vi "UHR-Fleezers Control (host) - Avogadro v1.vi"() -> ()   [LabVIEW 2014] (continued)
  out "GI Late Counter 2":u8
  in  "Phase adj. (GI) 2":i16=1
  out "GI relative phase 2":i16
  in  "+ phase (GI) 2":bool
  in  "Initial Phase Adjustment (GI) 2":i16=-274
  in  "- phase (GI) 2":bool
  in  "Green FB Gains":T14={"proportional gain (Kc)"=10, "integral gain (Kc*Ts/Ti)"=5, "derivative gain (Kc*Td/Ts)"=0}
  in  "Green int current ON count adj":u32=150
  in  "- phase (GI)":bool
  in  "Initial Phase Adjustment (GI)":i16=-28
  in  "+ phase (GI)":bool
  out "GI relative phase":i16
  in  "Phase adj. (GI)":i16=1
  out "GI Late Counter":u8
  out "Green AI Late Counter":u8
  out "MCL Scan":cluster{"Begin (V)":dbl, dbl, dbl[]}(graph)
  out "MCL Scan 2":cluster{"Begin (V)":dbl, dbl, dbl[]}(graph)
  out "Red laser intensity (V)":dbl
  out "Red AI Count":u16=600
  in  "Initial Phase Adjustment (RI)":i16=25
  out "RI Late Counter":u8
  in  "Red FB Gains":T14={"proportional gain (Kc)"=10, "integral gain (Kc*Ts/Ti)"=5, "derivative gain (Kc*Td/Ts)"=0}
  in  "Phase adj. (RI)":i16=20
  out "RI relative phase":i16
  in  "+ phase (RI)":bool
  in  "- phase (RI)":bool
  in  "Blue Laser Modulation Mode":string(combo)
  out "Digital Modulation":bool
  out "Analog Modulation":bool
  out "Laser On":bool
  in  "Get Blue Laser State":bool
  out "Blue laser intensity (V)":dbl
  out "Relative phase (BI AO)":i16
  out "Relative phase (BI DO)":i16
  out "Late Counter (BI DO)":u8
  out "Late Counter (BI AO)":u8
  in  "Initial Phase Adjustment (BI DO)":i16=65
  in  "Initial Phase Adjustment (BI AO)":i16
  in  "Phase adj. (BI AO)":i16=20
  in  "+ phase (BI AO)":bool
  in  "- phase (BI AO)":bool
  in  "Blue int AO ON count adjust":u16=150
  in  "Blue FB Gains":T14={"proportional gain (Kc)"=10, "integral gain (Kc*Ts/Ti)"=5, "derivative gain (Kc*Td/Ts)"=0}
  in  "- phase (BI DO)":bool
  in  "+ phase (BI DO)":bool
  in  "Phase adj. (BI DO)":i16=20
  out "Blue AI Count":u16=600
  in  "Delay (ms)":i32=500
  in  "Send string\nto Blue Laser":bool
  in  "command string":string
  out "command string sent":string="sames 0"
  out "read blue buffer":string
  out "Blue Error Out":errorcluster={"status"=TRUE, "code"=-1073807346, "source"="VISA Write in serial write macro.vi->UHR-Fleezers Control (host) - Avogadro v1.vi"}
  in  "VISA resource name":refnum<visa-resource-name>="Blue-Laser-COM7"
  in  "Blue Laser Modulation\nPower (mW)":string="80"
  in  "Blue Laser Power (mW)\n(Constant Power Mode)":string="70"
  in  "Flip X Sign":bool=TRUE
  in  "Trap Position FIFO Depth":u32=300000 format="%.0p"
  in  "# Samples/trap":u32=20000
  out "Trap AI Elements/DMA read":u32=320000 format="%.0p"
  out "Ave. Rate (Hz)":dbl=200000.0 format="%#_6p"
  out "FIFO El. Rem.":u32=3 format="%.0p"
  in  "Phase adj. (AI1)":i16=10
  out "Relative phase (AI1)":i16=-170
  in  "+ phase (AI1)":bool
  in  "- phase (AI1)":bool
  out "Late Counter (AI1)":u8
  in  "Initial Phase Adjustment (AI1)":i16=170
  out "AI rate (Hz)":dbl=200000.0 format="%#_6p"
  in  "AI Count (ticks)":u16=200
  out "# Samples/channel":u32=40000 format="%.0p"
  in  "Trap AI FIFO Depth":u32=900000
  in  "Detector Type":string(combo)="IR-QPD + PSD + FB-QPD X position"
  in  "N Acq Sets (Traps + Fl.)":i16=2
  in  "Sets to FIFO (Traps)":T22={"Set 1"=TRUE, "Set 2"=TRUE, "Set 3"=FALSE}
  in  "FPGA Ave.":dbl=1.0 min=1.0 step=1.0
  out "Ave. Period (s)":dbl=5e-06 format="%#_6p"
  out "DMA Update Period (s)":dbl=0.2
  out "FPGA Averaging":bool
  out "Trap Sets":u32=2
  out "Counts/DMA":dbl=8000000.0 format="%#_6p"
  out "Trap Pos FIFO El Remaining":u32=2905 format="%.0p"
  out "Trap Pos Elements/DMA read":u32=200000 format="%.0p"
  out "Trap AI FIFO Timeout":u16
  out "Trap Pos FIFO Timeout":u16
  out "error out":errorcluster
  out "error out 2":errorcluster
  in  "Piezo trap y\noffset (V)":dbl=0.6709036530655844
  in  "Piezo trap x\noffset (V)":dbl=-6.361797973205792
  in  "Piezo Trap Y cal (nm/V)":dbl=279.6
  in  "Piezo Trap X cal (nm/V)":dbl=362.7
  in  "Bottom  1 Harvard Syringe Pump Serial Port":refnum<visa-resource-name>="Bottom-Pump1-COM5"
  in  "Center Harvard Syringe Pump Serial Port":refnum<visa-resource-name>="Central-Pump2-COM6"
  in  "Lost Tether Alarm Threshold (pN)":dbl=0.5
  in  "AOM X Cal (nm/MHz)":dbl=203.0
  in  "MCL X Cal (nm/V)":dbl=739.5
  out "X RF Amplitude Limits (%)":T23={"Minimum"=0.0, "Maximum"=50.0, "Increment"=1.0}
  out "X RF Frequency Limits (MHz)":T23={"Minimum"=60.0, "Maximum"=90.0, "Increment"=1.0}
  out "Y RF Frequency Limits (MHz)":T23={"Minimum"=0.0, "Maximum"=40.0, "Increment"=0.1}
  out "Y RF Amplitude Limits (%)":T23={"Minimum"=0.0, "Maximum"=45.0, "Increment"=1.0}
  in  "Manip. X?":bool=TRUE
  in  "Manip. Y?":bool
  in  "Force Manip Abort":bool
  out "Read cal error":errorcluster
  in  "DAQ Delay (ms)":u32=1000
  in  "Start Scan":bool
  in  "Scan axis":bool=TRUE
  in  "Osc. amp. (V)":dbl=5.0
  in  "Osc. center (V)":dbl=5.0
  in  "Osc. freq. (Hz) 2":dbl=1.0
  in  "MCL Mode":u16(ring) items=["Manual Positioning", "Sinusoidal Wave", "Linear Scan"]
  in  "Begin (V)":dbl
  in  "End (V)":dbl=10.0
  in  "N Points":dbl=20.0
  in  "Delay to Interlace (s)":dbl
  in  "Delayed Interlace Start":bool
  in  "Read Lateness and Rel Phase":bool=TRUE
  out "Vec Mean of T1 T2":dbl[](array[numeric])=[-361.2890180339416, -361.0696389052203]
  in  "Cal read wait (s)":u32=5
  out "Time tether formed":timestamp=timestamp(3534521622.0325327 s since 1904-01-01)
  in  "Sample Chamber Stage Serial Port":refnum<visa-resource-name>="Sample-Stage-COM1"
  in  "Chemyx Syringe Pump Serial Port":refnum<visa-resource-name>="ASRL3::INSTR"
  in  "Limit Min (MHz)":dbl=10.0 caption="Min (MHz)"
  in  "Limit Max (MHz)":dbl=16.0 caption="Max (MHz)"
  in  "Limits Enable":bool=TRUE caption="Enable"
  out "AI labels":string[](array[string])=["T1 Y", "T1 X", "T1 Sum", "T2 Y", "T2 X", "T2 Sum", "T1 FB X", "T1 FB Sum", "T2 FB X", "T2 FB Sum", "T3 Y/ PSD Y", "T3 X / PSD X", "T3 Sum / PSD sum"]
  in  "Save Trap Pos. Data":bool=TRUE
  in  "Lower Ch. Cap.":bool
  in  "Top 3 Harvard Syringe Pump Serial Port":refnum<visa-resource-name>="Top-Pump3-COM4"
  out "Database link":path=path "C:/Home/Bustamante Lab/Comstock-LabView-Link.udl"
  out "connection reference":T24
  out "FPGA error out":errorcluster
  out "Trigger Signal":dbl[](graph)=[1.953852737276498, 1.8613052147403675]
  in  "Fish mask thresh":dbl=0.5
  in  "Normal (on) or masked test (off)":bool=TRUE
  in  "Stop F (pN) (mask)":dbl=1.0
  in  "Osc. freq. (Hz)":dbl=0.25
  in  "Trap shift\nmethod":bool=TRUE
  in  "Pause rotation":bool
  out "Waveform Chart":dbl(graph)
  in  "Trap 2 phase shift (deg)":dbl caption="Fixed phase shift (deg)"
  in  "Radius (MHz)":dbl=2.0 min=0.0 max=10.0 step=0.1
  out "Trap trajectories":cluster{dbl[], dbl[]}[](graph)
  in  "Move in a Circle":bool
  in  "Center Y Frequency (MHz)":dbl=31.0
  in  "Stop Moving":bool
  in  "2D Motion Frequency (Hz)":dbl=0.25
  in  "2D Motion Trap Separation (MHz)":dbl=0.75 caption="Fixed distance (MHz)" min=0.0 max=10.0 step=0.1
  in  "Time step (ms)":i64=10
  in  "N steps then stop":i32
  in  "Back to start on finish?":bool=TRUE
  in  "Counterclockwise/Clockwise":bool
  out "Trap 1 sum mean":dbl=-0.0915169228862244 format="%0.2f"
  out "Trap 2 sum mean":dbl=-0.06760925671124465 format="%0.2f"
  in  "index 1":i32=3
  in  "index 2":i32
  in  "test":bool
  in  "Reset graph":bool
  in  "N steps to plot":i32=1000
  out "Waveform Graph 2":waveform(dbl)(graph)
  in  "Offset 2":dbl
  in  "mult x":dbl
  in  "Offset":dbl
  out "N data samples":dbl
  out "Initial buffer time (s)":dbl
  in  "N initial buffer elements":u16=5000
  in  "Sound ON":bool
  in  "Carrier Frequency (Hz)":dbl=300.0
  in  "number of samples/ch":i32=100000
  in  "sample mode":T25=1 items=["Finite Samples", "Continuous Samples"]
  in  "device ID":u32
  in  "sound format":T26={"sample rate (S/s)"=22050.0, "number of channels"=2, "bits per sample"=16}
  in  "Volume":dbl=1.0 format="%0.2p"
  in  "interpolation mode":u16(ring)=1 items=["coerce", "linear", "spline", "FIR filter"]
  in  "tone or data":bool
  in  "Data channel to sound":i32
  in  "Base N trap periods":u32=50
  in  "Period scale factor":dbl=4.0
  in  "Trap osc amp (MHz)":dbl=1.0
  in  "Osc trap cont.":bool
  in  "Osc traps":bool
  out "Trap OSC Period (s)":dbl=0.002
  out "Writing waveform to fpga memory":bool
  in  "Save trap pos with cal":bool=TRUE
  in  "T1 Osc Enable":bool=TRUE
  in  "T2 Osc Enable":bool=TRUE
  out "DMA remainder":u64
  out "(total save/100) /osc period remainder":u32
  out "Total save/100 remainder":u32
  out "N osc/ (total save/100)":u64=25
  out "N osc / DMA":u64=100
  out "N trap osc periods per save":u64
  out "N trap osc periods per save remainder":u64
  in  "Command":string
  out "Reply":string
  in  "Send Command":bool
  out "Preamp Error Out":errorcluster
  in  "Gain Mode":string(combo)="0"
  in  "Invert Signal":bool
  in  "Sensitivity":string(combo)="0"
  in  "Offset Current Sign":bool=TRUE
  in  "Offset Current Value":string(combo)
  in  "Offset Current":bool
  in  "Bias Voltage":bool
  in  "Bias Voltage (mV)":i32
  in  "Filter Type":string(combo)="4"
  in  "Lowpass 3dB Point":string(combo)="6"
  in  "Highpass 3dB Point":string(combo)
  in  "Filter Reset":bool
  out "Command Sent":string
  out "Gain":string(combo)="0"
  # "X"
  # "Y"
  # "Data Saving"
  # "External fluorescence triggering tests:"
  # "After"
  # "During"
  # "Trap On?"
  # "BD Flow ON?"
  # "Samp Flow ON?"
  # "Trap Trig. Fl.?"
  # "Zero It"
  # "Floor it\n(e.g., hp unwinding)"
  # "1"
  # "2"
  # "Fl. Down"
  # "Fl. Up"
  # "T1 Y"
  # "T1 X"
  # "T1 Sum"
  # "T2 Y"
  # "T2 X"
  # "T2 Sum"
  # "FB1 X"
  # "FB1 Sum"
  # "FB2 X"
  # "FB2 Sum"
  # "T3 Y"
  # "T3 X"
  # "T3 Sum"
  # "Trap Display:"
  # "APD Display:"
  # "DAQ"
  # "Trap Manipulation"
  # "Bead Calibration"
  # "MCL trap"
  # "Trap 3"
  # "Fl"
  # "Fine Motor Control"
  # "Bottom Pump (#1)"
  # "Central Sample Channels"
  # "Top Pump (#3)"
  # "Rate param is ul/h\nVolume param is ul"
  # "Chemyx Pump 2"
  # "Units: \n1 = ml/m\n2 = ml/h\n3 = ul/m\n4 = ul/h"
  # "Choose method of updating trap RF values: false is usual, true is use external loop method\n(in order to increase possible delay between X and Y signals -- to synchronize X and Y switching)"
  # "Delay to switch frequency and amplitude of boards.\nUsed to align phases of boards (finely)."
  # "X"
  # "Y"
  # "Oscillate Set 1 freq. (debugging)"
  # "BD 1"
  # "BD 2"
  # "Amp switch 1st is disabled in the fpga!\nSeems its also frequency that needs to go first (for all boards tested so far)."
  # "AOD Raster Scan"
  # "Approx. trap separations"
  # "X"
  # "Y"
  # "FPGA\nreading"
  # "DMA\ntransfer"
  # "APD Integration Loop"
  # "APD Gates"
  # "APD 2 (Cy5)"
  # "APD 3 (Cy2)"
  # "APD 1 (Cy3)"
  # "X"
  # "2D"
  # "Y"
  # "1D"
  # "Digital Out Control"
  # "Analog Out Control (Feedback Loop)"
  # "Laser Intensity Analog Input"
  # "Operational note:\n\nUse the digital out control to adjust red laser\ntiming (fine tuning).\n\nAt the moment, the red laser analog out\ncontrol timing is identical and set by green \nlaser AO timing (in the same loop).  Otherwise\nyou can not get synchronous timing with the\ncurrent AO expansion board.\n\nSimilarly, the AI measurement is also \nsimultaneous for all three lasers (for the same\nreason).\n\nThese controls are kept for possible future\nuse."
  # "Analog Out Control (Feedback Loop)"
  # "Digital Out Control"
  # "Laser Intensity Analog Input"
  # "Operational note:\n\nThe AI measurement is simultaneous for all three lasers\n(see red laser note).\n\nThese controls are kept for possible future use."
  # "Analog Out Control (Feedback Loop)"
  # "Laser Intensity Analog Input"
  # "Digital Out Control"
  # "Total AI Rates (NOT rates/trap)"
  # "(Samples/trap x Trap Sets)"
  # "(Samples/channel x\n8 if averaging (8 channels)\n4 if no averaging)"
  # "Trap 1"
  # "Trap 2"
  # "Flour./Trap 3"
  # "External Video Window"
  # "3: IR LED\n2: Blue LED"
  # "MCL Position Debugging"
  # "Temporary Control Storage\n(these used to be somewhere else, still want to keep them)"
  # "Database config"
  # "Y"
  # "X"
  # "Trap Position Difference Limits"
  # "Start trapping above center (> center MHz)\n\nNegative trap separation means trap 2 follows\n(starts to the right)"
  # "Initialization"
  # "Radius initially determined by center\nand current location (then can be changed)"
  # "Active (oscillating) trap calibration:"
  # "All these remainders\nshould be 0."
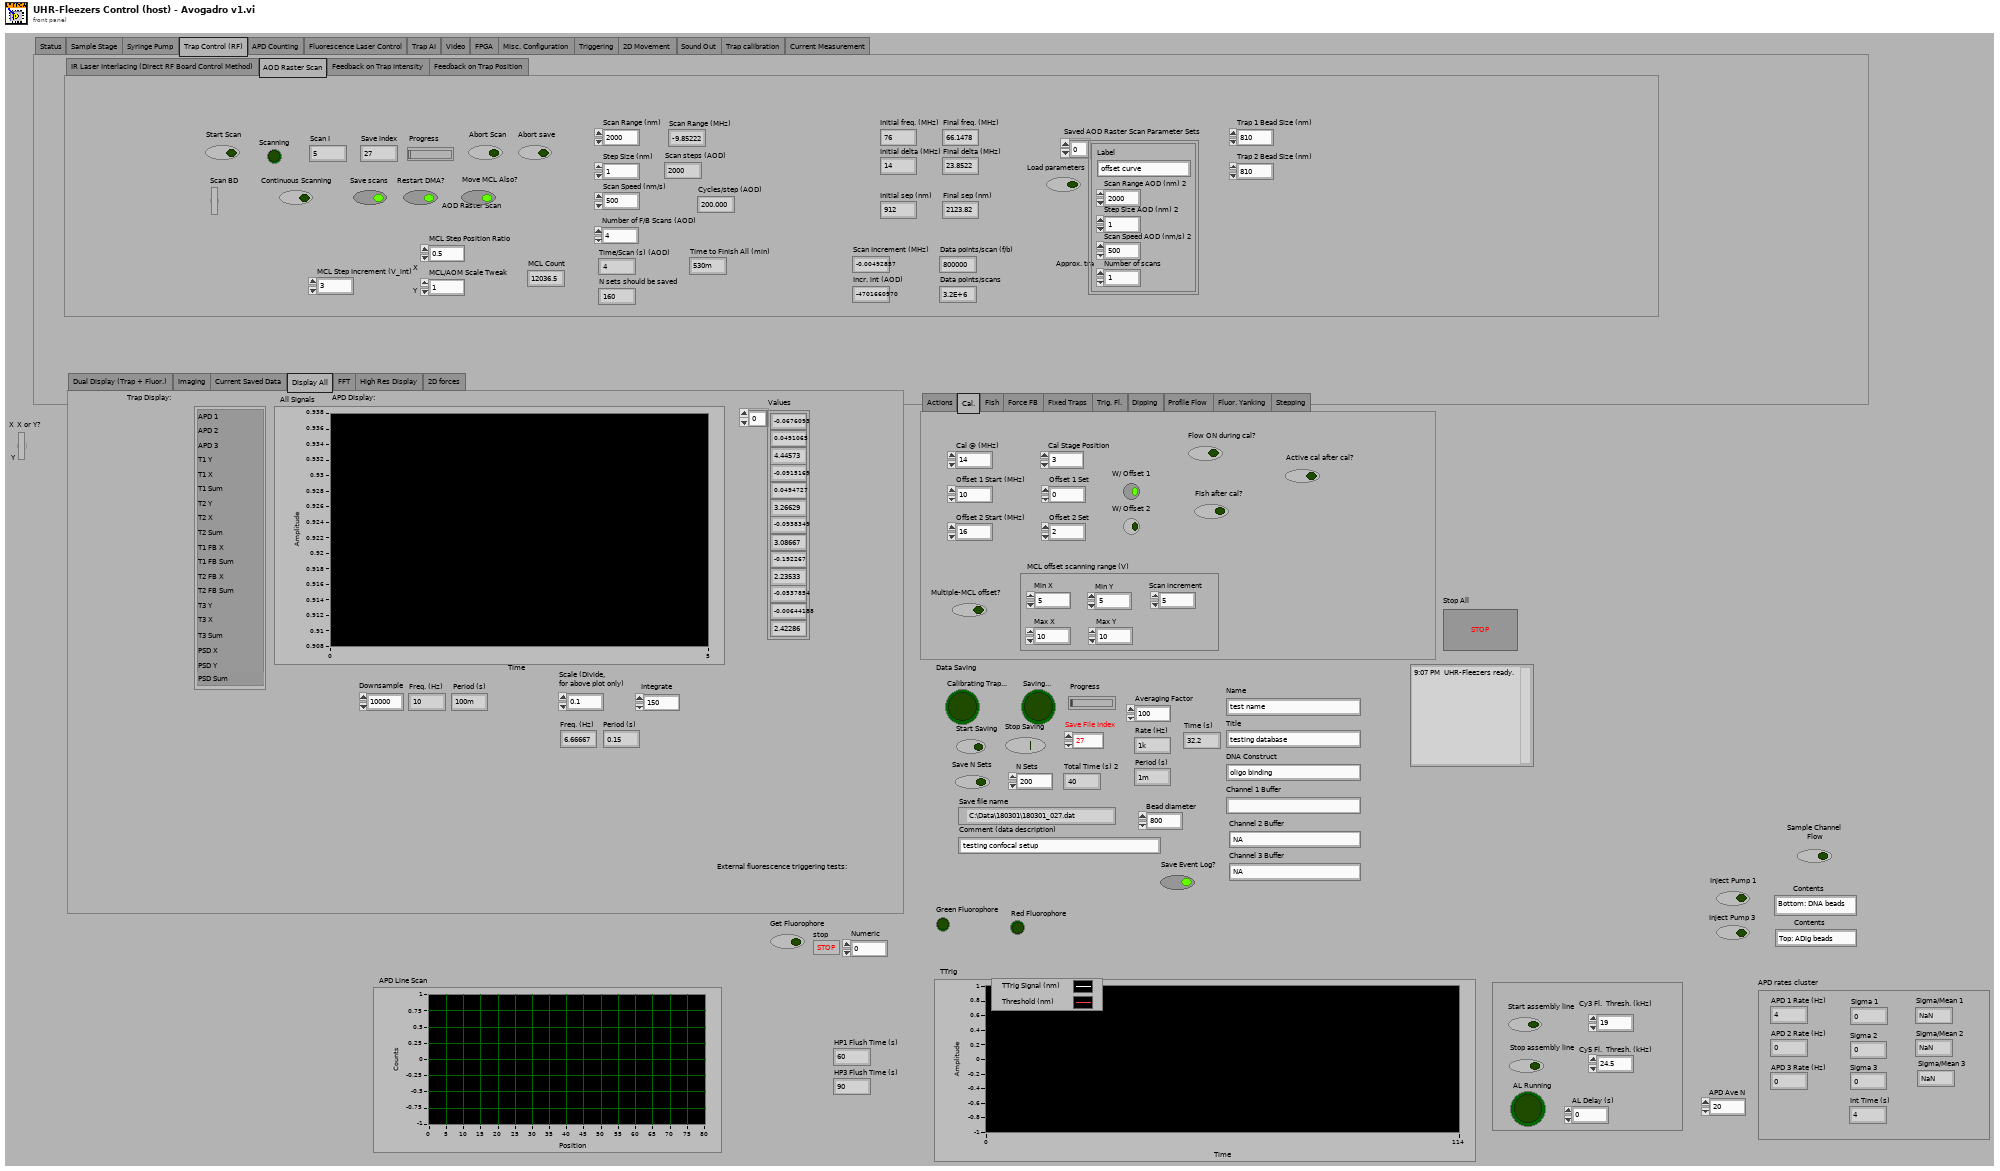
[diagram p1: front panel]
types:
  T1 = cluster{"APD 1 Rate (Hz)":dbl, "APD 2 Rate (Hz)":dbl, "APD 3 Rate (Hz)":dbl, "Sigma/Mean 1":dbl, "Int Time (s)":dbl, "Sigma 1":dbl, "Sigma 2":dbl, "Sigma 3":dbl, "Sigma/Mean 2":dbl, "Sigma/Mean 3":dbl}
  T2 = enum32{"Actions", "Cal.", "Fish", "Force FB", "Fixed Traps", "Trig. Fl.", "Dipping", "Profile Flow", "Fluor. Yanking", "Stepping"}
  T3 = cluster{"Min X":u32, "Max X":u32, "Min Y":u32, "Max Y":u32, "Scan increment":dbl}
  T4 = enum32{"Dual Display (Trap + Fluor.)", "Imaging", "Current Saved Data", "Display All", "FFT", "High Res Display", "2D forces"}
  T5 = cluster{"T1 X":dbl, "T2 X":dbl, "T3 X":dbl, "T3 Y":dbl}
  T6 = cluster{"T1 X":bool, "T2 X":bool, "T3 X":bool, "T3 Y":bool}
  T7 = typedef "IMAQ Image.ctl" = refnum<image>
  T8 = enum32{"Status", "Sample Stage", "Syringe Pump", "Trap Control (RF)", "APD Counting", "Fluorescence Laser Control", "Trap AI", "Video", "FPGA", "Misc. Configuration", "Triggering", "2D Movement", "Sound Out", "Trap calibration", "Current Measurement"}
  T9 = cluster{"alpha_x (nm/V)":dbl, "offset_x (mV)":dbl, "kappa_x (pN/nm)":dbl, "alpha_y (nm/V)":dbl, "kappa_y (pN/nm)":dbl, "offset_y (mV)":dbl}
  T10 = cluster{"Pump 1":cluster{"Diameter (mm)":dbl, "Units":dbl, "Volume":dbl, "Rate":dbl}, "Pump 2":cluster{"Diameter (mm)":dbl, "Units":dbl, "Volume":dbl, "Rate":dbl}, "Pump 3":cluster{"Diameter (mm)":dbl, "Units":dbl, "Volume":dbl, "Rate":dbl}}
  T11 = enum32{"IR Laser Interlacing (Direct RF Board Control Method)", "AOD Raster Scan", "Feedback on Trap Intensity", "Feedback on Trap Position"}
  T12 = typedef "LVPoint32TypeDef.ctl" = cluster{"Horizontal":i32, "Vertical":i32}
  T13 = cluster{"Scan Range AOD (nm) 2":dbl, "Step Size AOD (nm) 2":dbl, "Scan Speed AOD (nm/s) 2":dbl, "Number of scans (AOD) 2":u16, "Label":string}[]
  T14 = cluster{"proportional gain (Kc)":i16, "integral gain (Kc*Ts/Ti)":i16, "derivative gain (Kc*Td/Ts)":i16}
  T15 = cluster{"Trap 1":fxp<+/-,16,1>, "Trap 2":fxp<+/-,16,1>}
  T16 = enum32{"Main Setting", "Details", "Dynamic FB settings", "Semi Passive Mode"}
  T17 = cluster{"proportional gain (Kc)":fxp<+/-,16,8>, "integral gain (Kc*Ts/Ti)":fxp<+/-,16,8>, "derivative gain (Kc*Td/Ts)":fxp<+/-,16,8>}
  T18 = cluster{"output high":fxp<+/-,16,1>, "output low":fxp<+/-,16,1>}
  T19 = cluster{"Set 1":fxp<+/-,16,1>, "Set 2":fxp<+/-,16,1>}
  T20 = cluster{"Trap 1X offset":dbl[], "Trap 2X offset":dbl[]}
  T21 = enum32{"Main Controls", "Green laser (532 nm)", "Red laser (633 nm)", "Blue laser (473 nm)"}
  T22 = cluster{"Set 1":bool, "Set 2":bool, "Set 3":bool}
  T23 = typedef "LVMinMaxIncTypeDef.ctl" = cluster{"Minimum":dbl, "Maximum":dbl, "Increment":dbl}
  T24 = typedef "NI_Database_API.lvlib/Conn ObjectReference.ctl" = refnum<k1>
  T25 = typedef "Sampling Mode.ctl" = i32
  T26 = typedef "Sound Data Format.ctl" = cluster{"sample rate (S/s)":dbl, "number of channels":i32, "bits per sample":i32}
  T27 = typedef "nirio_resource_hc.ctl" = tag
  T28 = typedef "Image Type" = u32
  T29 = typedef "Pressure Control.lvclass/Pressure Control Config.ctl" = cluster{"daqmx_channel":string, "terminal_configuration":string}
  T30 = cluster{string, "TTL line # Pressure Up":u8, bool, bool}
  T31 = cluster{string, "TTL line # Pressure Down":u8, bool, bool}
  T32 = cluster{string, "TTL line # Pressure Vacuum":u8, bool, bool}
  T33 = cluster{string, "TTL line # Pressure Vacuum":u8, bool, bool}[]
  T34 = cluster{"New Image":T7, "New Image":T7, "New Image":T7, "New Image":T7, "New Image":T7}
  T35 = typedef "XDNodeRunTimeDep.lvlib/timing_clust.ctl" = cluster{"Expected End [f-1]":u64, "Actual End [f-1]":u64, "Finished Late? [f-1]":bool, "Expected End [i-1]":u64, "Actual End [i-1]":u64, "Finished Late? [i-1]":bool, "Expected Start [i]":u64, "Actual Start [i]":u64, "Expected Start [f]":u64, "Actual Start [f]":u64, "Source Name":string, "Structure Name":string, "Period":i64, "Deadline":i64, "Offset":i64, "Start":i64, "Priority":i32, "Timeout":i32, "Mode":T36, "Wakeup Reason":T37, "Error":errorcluster, "Source Type":string, "Secondary Source Type":string, "Global End Time":u64, "Global Start Time":u64, "Frame Duration":u64, "Iteration Duration":u64, "Assigned CPU":i32, "I/O Scan Engine Mode":u32}
  T36 = typedef "XDNodeRunTimeDep.lvlib/nitl_modes.ctl" = enum32{"No Change", "Process missed periods, maintain original phase", "Discard missed periods, maintain original phase", "Process missed periods, ignore original phase", "Discard missed periods, ignore original phase"}
  T37 = typedef "XDNodeRunTimeDep.lvlib/wakeup.ctl" = enum32{"Normal", "Aborted", "Asynchronous wakeup", "Timing source error", "Timed loop error", "Timeout"}
  T38 = enum16{"Trackball XY", "Trackball Z", "Trackball OFF", ""}
  T39 = enum32{"Status", "Sample Stage", "Syringe Pump", "Trap Control (RF)", "APD Counting", "Fluorescence Laser Control", "Trap AI", "Video", "FPGA"}
  T40 = enum32{"Status", "Sample Stage", "Syringe Pump", "Trap Control (RF)", "APD Counting", "Fluorescence Laser Control", "Trap AI", "Video", "FPGA", "Misc. Configuration"}
  T41 = typedef "openfpgaref.8.6.ctl" = refnum<k20>
  T42 = enum16{"CONNECT", "INITIALIZE VALVES", "DISCONNECT", "MOVE VALVE"}
  T43 = enum16{"empty", "write", "read oldest (queue)", "read newest (stack)", "read all"}
  T44 = enum16{"open", "replace", "create", "open or create", "replace or create", "replace or create with confirmation"}
  T45 = enum16{"big-endian, network order", "native, host order", "little-endian"}
  T46 = cluster{"Scan Range AOD (nm) 2":dbl, "Step Size AOD (nm) 2":dbl, "Scan Speed AOD (nm/s) 2":dbl, "Number of scans (AOD) 2":u16, "Label":string}
  T47 = cluster{"alpha_x (nm/V)":dbl, "offset_x (mV)":dbl, "kappa_x (pN/nm)":dbl, "alpha_y (nm/V)":dbl, "kappa_y (pN/nm)":dbl, "offset_y (mV)":dbl}[]
  T48 = cluster{"[0]":dbl, "[1]":dbl, "[2]":dbl, "[3]":dbl, "[4]":dbl, "[5]":dbl}
  T49 = cluster{"Diameter (mm)":dbl, "Units":dbl, "Volume":dbl, "Rate":dbl}
  T50 = cluster{"Left":i32, "Top":i32, "Width":u32, "Height":u32}
  T51 = cluster{cluster{"Left":i32, "Top":i32, "Width":u32, "Height":u32}}[]
  T52 = typedef "Sound Output Task ID.ctl" = u32
  T53 = enum32{"Normal Display", "Dual Display (APD)", "FFT", "High Res Display"}
  T54 = cluster{"Origin Pixel":cluster{"X":sgl, "Y":sgl}, "Angle Relative to Horizontal (deg)":sgl, "Axis Reference":u32}
  T55 = typedef "Simple Grid Descriptor" = cluster{"X Step":sgl, "Y Step":sgl, "Unit":T56}
  T56 = typedef "Image Unit" = enum32{"Undefined", "Angström", "Micrometer", "Millimeter", "Centimeter", "Meter", "Kilometer", "Microinch", "Inch", "Feet", "Nautical miles", "Standard miles", "Steps"}
  T57 = enum32{"Dual Display (Trap + Fluor.)", "Imaging", "Current Saved Data", "Display All", "FFT", "High Res Display"}
  T58 = cluster{"averaging mode":u16, "weighting mode":u16, "number of averages":u32}
  T59 = cluster{"dB On (F)":bool, "unwrap phase (F)":bool, "convert to degree (F)":bool}
  T60 = cluster{"Scan Range (nm)":dbl, "MCL Step Position Ratio":dbl, "MCL/AOM Scale Tweak":dbl, "MCL X Cal (nm/V)":dbl, "MCL Step Increment (V_int)":dbl, "Total Counts (ticks)":u16, "Scan steps (AOD)":u64, "Cycles/step (AOD)":u64}
  T61 = cluster{"Actual MCL Inc (V)":dbl, "Scan steps (MCL)":u64, "Scan lines (y)":u64, "AO1":dbl, "AO2":dbl}
  T62 = cluster{"Actual MCL Inc (V)":dbl, "Scan steps (MCL)":u64, "Scan lines (y)":u64, "T3 Y (V)":dbl, "T3 X (V)":dbl}
  T63 = cluster{"APD 1":u32[], "APD 2":u32[], "APD 3":u32[]}
  T64 = cluster{"RMS[0]":dbl, "RMS[1]":dbl, "RMS[2]":dbl, "RMS[3]":dbl}
  T65 = cluster{"Mean [0]":dbl, "Mean [1]":dbl, "Mean [2]":dbl, "Mean [3]":dbl}
  T66 = cluster{"f0":dbl, "df":dbl, "magnitude":dbl[]}[][]
  T67 = cluster{"Comment (data description)":string, "Channel 1 Buffer":string, "Channel 2 Buffer":string, "Channel 3 Buffer":string, "Title":string, "DNA Construct":string, "Bead diameter":dbl, "Name":string}
diagram:
  w9 = 90.0
  w36 = T28 2 items=["Grayscale (U8)", "Grayscale (I16)", "Grayscale (SGL)", "Complex (CSG)", "RGB (U32)", "HSL (U32)", "RGB (U64)", "Grayscale (U16)"] ("Image Type")
  # "Stage controller reference"
  # "X limits"
  # "Amp Lmits"
  # "Freq Limits"
  # "Changed by Ronen - All events relating to activation of the pumps have been disabled: 56, 55, 54, 53, 52, 51, 50, 49, 48, 47, 46, 45, 44, 43, 41, 40"
  # "Harvard Pump control disabled by Hendrik"
  # "Settings to help prevent AOM/D damage"
  # "Initialize the FPGA DAQ card itself"
  # "Reset the DAQ card."
  # "Specify the DAQ card and the FPGA code to run"
  # "Bottom 1 Harvard"
  # "Top 3 Harvard"
  # "Center Harvard"
  n1 = disable-structure shown="Enabled" {
    frame Enabled {
      w105 = FALSE
      # "This Control added by\nRonen to enable direct\nControl of pressure pulse\nlength to enable fine flow\ncontrol"
      # "Start out with all lines set to zero"
      n2 = Format Into String(format string="%s/port0/line5:1, %s/port1/line0:3", "DAQmx Device Name", "DAQmx Device Name") -> (resulting string=w97:string)  [unwired: 2 in, 1 out]
      n3 = Format Into String(format string="%s/ai0", "DAQmx Device Name") -> (resulting string=w95:string)  [unwired: 2 in, 1 out]
      n4 = In Range and Coerce(upper limit=100.0, x="Pulse Duration (0-100 ms)", lower limit=0.0) -> (coerced(x)=w80:dbl)  [unwired: 1 out]
      n5 = Bundle By Name(cluster=T29 {"daqmx_channel"="", "terminal_configuration"=""} ("Pressure Control Config"), "daqmx_channel"=w95, "terminal_configuration"="RSE") -> (w112:T29)
      n6 = To Unsigned Long Integer(number=w80) -> (unsigned 32bit integer=w79:u32)
      n7 = Bundle("Pressure up", "TTL line # Pressure Up"=u8 6, w105, w105) -> (w103:T30)  [unwired: 1 in]
      n8 = Bundle("Pressure down", "TTL line # Pressure Down"=u8 8, w105, w105) -> (w104:T31)  [unwired: 1 in]
      n9 = Bundle("Pressure vacuum", "TTL line # Pressure Vacuum"=u8 7, w105, w105) -> (w102:T32)  [unwired: 1 in]
      n10 = Build Array(w103, w104, w102) -> (w101:T33)
      n11 = call "Initialize.vi"("Pulse duration (ms)"=w79, "TTL Ports"=w97, "TTL in"=refnum<class "TTL.lvclass"> refnum ("TTL.lvclass")) -> ("error out"=w100:errorcluster, "TTL out"=w89:refnum<class "TTL.lvclass">)  [unwired: 7 in]
      n12 = call "Initialize.vi"("TTL Lines"=w101, "error in (no error)"=w100, "TTL"=w89, "Pressure Control Config"=w112, "Pressure Control in"=refnum<class "Pressure Control.lvclass"> refnum ("Pressure Control.lvclass")) -> ("error out"=w117:errorcluster, "Pressure Control out"=w99:refnum<class "Pressure Control.lvclass">)  [unwired: 5 in]
      n13 = call "Get line states.vi"("error in (no error)"=w117, "TTL in"=w89) -> ("error out"=w84:errorcluster, "Current line states"=w85:bool[], "TTL out"=w88:refnum<class "TTL.lvclass">)  [unwired: 7 in]
      n14 = Array Size(array=w85) -> (size(s)=w86:i32)
      n15 = for {
        N: w86 -> [_]
        shift-right: [w123] -> w87
        shift-left: w88 -> [w124]
        shift-right: [w121] -> w118
        shift-left: w84 -> [w122]
        i -> [w120]
        n16 = call "Set line.vi"("error in (no error)"=w122, "Action"=enum16{"Open", "Close", "Toggle"}."Open", "Line number"=w120, "TTL in"=w124) -> ("error out"=w121:errorcluster, "TTL out"=w123:refnum<class "TTL.lvclass">)  [unwired: 6 in]
      }
      n17 = case shown="No Error" w118 {
        selector: w118 -> [_ w178]
        tunnel: w99 -> [w129 _]
        tunnel: w87 -> [w128 _]
        tunnel: [w125 w177] -> w92
        frame No Error {
          n18 = while {
            shift-right: [w137] -> w126
            shift-left: w129 -> [w136]
            shift-right: [w135] -> w127
            shift-left: w128 -> [w134]
            stop <- w132 stop-if-true
            n19 = call "Get pressure.vi"("Pressure Control in"=w136) -> ("Pressure"=→"Pressure":dbl)  [unwired: 7 in, 3 out]
            n20 = event shown="[7] \"Pulse Duration (0-100 ms)\": Value Change" {
              selector: _ -> [_ _ _ _ _ _ _ _]
              dyn-events: _ -> [_ _ _ _ _ _ _ _]
              timeout: 100 -> [_ _ _ _ _ _ _ _]
              tunnel: [w140 w143 w144 w149 w153 w158 w163 w175] -> w137
              tunnel: w136 -> [w140 w143 w145 w150 w154 w159 w164 w176]
              tunnel: [w139 w142 w146 w151 w155 w160 w165 w173] -> w135
              tunnel: w134 -> [w139 w142 w146 w151 w155 w160 w165 w174]
              tunnel: [_ TRUE _ _ _ _ _ _] -> w132
              tunnel: [_ _ w147 w152 w156 w161 w166 w172] -> w131
              event Timeout {
                n21 = event-data() -> ()  [unwired: 1 in, 2 out]
              }
              event "Stop All": Value Change {
                n22 = event-data() -> ()  [unwired: 1 in, 6 out]
              }
              event "Vent pressure": Value Change {
                n23 = event-data() -> ()  [unwired: 1 in, 5 out]
                n24 = call "Vent.vi"("Pressure Control in"=w145) -> ("error out"=w147:errorcluster, "Pressure Control out"=w144:refnum<class "Pressure Control.lvclass">)  [unwired: 9 in]
              }
              event "Vacuum": Value Change {
                n25 = event-data() -> ("NewVal"=w148:bool)  [unwired: 1 in, 4 out]
                n26 = call "Set vacuum.vi"("Vacuum?"=w148, "Pressure Control in"=w150) -> ("error out"=w152:errorcluster, "Pressure Control out"=w149:refnum<class "Pressure Control.lvclass">)  [unwired: 8 in]
              }
              event "Set zero pressure": Value Change {
                n27 = event-data() -> ()  [unwired: 1 in, 5 out]
                n28 = call "Set zero pressure to current pressure.vi"("Pressure Control in"=w154) -> ("error out"=w156:errorcluster, "Pressure Control out"=w153:refnum<class "Pressure Control.lvclass">)  [unwired: 8 in, 1 out]
              }
              event "Pressure Up": Value Change {
                n29 = event-data() -> ()  [unwired: 1 in, 5 out]
                n30 = call "Pressure pulse.vi"("Up or down?"=enum16{"Up", "Down"}."Up", "Pressure Control in"=w159) -> ("error out"=w161:errorcluster, "Pressure Control out"=w158:refnum<class "Pressure Control.lvclass">)  [unwired: 8 in]
              }
              event "Pressure Down": Value Change {
                n31 = event-data() -> ()  [unwired: 1 in, 5 out]
                n32 = call "Pressure pulse.vi"("Up or down?"=enum16{"Up", "Down"}."Down", "Pressure Control in"=w164) -> ("error out"=w166:errorcluster, "Pressure Control out"=w163:refnum<class "Pressure Control.lvclass">)  [unwired: 8 in]
              }
              event "Pulse Duration (0-100 ms)": Value Change {
                # "Event added by Ronen to allow for changes\nin pulse duration as program is running"
                n33 = event-data() -> ()  [unwired: 1 in, 6 out]
                n34 = local read "Pulse Duration (0-100 ms)"() -> (w170:dbl)
                n35 = In Range and Coerce(upper limit=100.0, x=w170, lower limit=0.0) -> (coerced(x)=w168:dbl)  [unwired: 1 out]
                n36 = To Unsigned Long Integer(number=w168) -> (unsigned 32bit integer=w167:u32)
                n37 = call "Change TTL - Ronen.vi"("Pulse Duration (ms)"=w167, "TTL.lvclass"=w174) -> ("error out"=w172:errorcluster, "TTL.lvclass"=w173:refnum<class "TTL.lvclass">)  [unwired: 8 in]
                n38 = call "Update TTL - Ronen.vi"("TTL.lvclass"=w173, "Pressure Control in"=w176) -> ("Pressure Control out"=w175:refnum<class "Pressure Control.lvclass">)  [unwired: 8 in, 1 out]
              }
            }
            n39 = call <vilib>:"Simple Error Handler.vi"("error in (no error)"=w131) -> ()  [unwired: 4 in, 5 out]
          }
          n40 = call "Close.vi"("Pressure Control in"=w126) -> ("error out"=w130:errorcluster)  [unwired: 9 in, 1 out]
          n41 = call "Close.vi"("error in (no error)"=w130, "TTL in"=w127) -> ("error out"=w125:errorcluster)  [unwired: 8 in, 1 out]
        }
        frame Error {
          n42 = call <vilib>:"Simple Error Handler.vi"("error in (no error)"=w178) -> ("error out"=w177:errorcluster)  [unwired: 4 in, 4 out]
        }
      }
      n43 = property on="DAQmx Device Name" class="DAQmxName"("Visible"=FALSE) -> ()  [unwired: 2 in, 2 out]
      n44 = call <vilib>:"Clear Errors.vi"("error in (no error)"=w92) -> ("error out"=w90:errorcluster)  [unwired: 5 in, 1 out]
      n45 = property on="DAQmx Device Name" class="DAQmxName"(error in=w90, "Visible"=TRUE) -> ()  [unwired: 1 in, 2 out]
    }
    frame Disabled {
    }
  }
  n46 = disable-structure shown="Disabled" {
    disable-tunnel: [w205 _] -> w48
    disable-tunnel: [w204 _] -> w47
    disable-tunnel: [w199 _] -> w43
    disable-tunnel: [w198 _] -> w42
    disable-tunnel: [w197 _] -> w41
    disable-tunnel: [w196 _] -> w40
    disable-tunnel: [w193 _] -> w32
    disable-tunnel: [w183 _] -> w13
    disable-tunnel: [w180 _] -> w12
    frame Disabled {
      w182 = u16 20 items=["1.0"=10, "1.5"=15, "2.0"=20] ("stop bits (10: 1 bit)")
      w191 = u16 20 items=["1.0"=10, "1.5"=15, "2.0"=20] ("stop bits (10: 1 bit)")
      w194 = u16 10 items=["1.0"=10, "1.5"=15, "2.0"=20] ("stop bits (10: 1 bit)")
      w200 = u16 20 items=["1.0"=10, "1.5"=15, "2.0"=20] ("stop bits (10: 1 bit)")
      w202 = u16 20 items=["1.0"=10, "1.5"=15, "2.0"=20] ("stop bits (10: 1 bit)")
      w206 = u16 20 items=["1.0"=10, "1.5"=15, "2.0"=20] ("stop bits (10: 1 bit)")
      # "Bottom 1 Harvard"
      # "Top 3 Harvard"
      # "Center Harvard"
      n47 = call-poly "VISA Configure Serial Port"("VISA resource name"=refnum<visa-resource-name> "COM2", "baud rate (9600)"=u32 9600, "stop bits (10: 1 bit)"=w191) -> ("VISA resource name out"=w183:refnum<visa-resource-name>, "error out"=→"Preamp Error Out":errorcluster)  [unwired: 4 in, 7 out]
      n48 = call-poly "VISA Configure Serial Port"("VISA resource name"=refnum<visa-resource-name> "COM2", "baud rate (9600)"=u32 9600, "stop bits (10: 1 bit)"=w182) -> ("VISA resource name out"=w180:refnum<visa-resource-name>)  [unwired: 4 in, 8 out]
      n49 = call-poly "VISA Configure Serial Port"("VISA resource name"=refnum<visa-resource-name> "COM7", "baud rate (9600)"=u32 115200, "stop bits (10: 1 bit)"=w194) -> ("VISA resource name out"=w193:refnum<visa-resource-name>, "error out"=w192:errorcluster)  [unwired: 4 in, 7 out]
      n50 = call-poly "VISA Configure Serial Port"("VISA resource name"=refnum<visa-resource-name> "COM5", "baud rate (9600)"=u32 115200, "stop bits (10: 1 bit)"=w200) -> ("VISA resource name out"=w197:refnum<visa-resource-name>, "error out"=w196:errorcluster)  [unwired: 4 in, 7 out]
      n51 = call-poly "VISA Configure Serial Port"("VISA resource name"=refnum<visa-resource-name> "COM4", "baud rate (9600)"=u32 115200, "stop bits (10: 1 bit)"=w202) -> ("VISA resource name out"=w199:refnum<visa-resource-name>, "error out"=w198:errorcluster)  [unwired: 4 in, 7 out]
      n52 = call-poly "VISA Configure Serial Port"("VISA resource name"=refnum<visa-resource-name> "COM6", "baud rate (9600)"=u32 115200, "stop bits (10: 1 bit)"=w206) -> ("VISA resource name out"=w204:refnum<visa-resource-name>, "error out"=w205:errorcluster)  [unwired: 4 in, 7 out]
      n53 = local write "Blue Error Out"(w192) -> ()
    }
    frame Enabled {
    }
  }
  n54 = call "IMAQ Create"("Image Name"="APD 1 Image", "Image Type"=w36) -> ("New Image"=w53:T7)  [unwired: 3 in, 1 out]
  n55 = call "IMAQ Create"("Image Name"="APD 2 Image", "Image Type"=w36) -> ("New Image"=w52:T7)  [unwired: 3 in, 1 out]
  n56 = call "IMAQ Create"("Image Name"="APD 3 Image", "Image Type"=w36) -> ("New Image"=w35:T7)  [unwired: 3 in, 1 out]
  n57 = call "IMAQ Create"("Image Name"="Det. X Image", "Image Type"=w36) -> ("New Image"=w51:T7)  [unwired: 3 in, 1 out]
  n58 = call "IMAQ Create"("Image Name"="Det. Y Image", "Image Type"=w36) -> ("New Image"=w50:T7)  [unwired: 3 in, 1 out]
  n59 = Bundle("New Image"=w53, "New Image"=w52, "New Image"=w35, "New Image"=w51, "New Image"=w50) -> (w49:T34)  [unwired: 1 in]
  n60 = call-poly "VISA Configure Serial Port"("VISA resource name"=refnum<visa-resource-name> "COM5", "timeout (10sec)"=u32 1000, "baud rate (9600)"=u32 19200) -> ("VISA resource name out"=w1:refnum<visa-resource-name>, "error out"=w4:errorcluster)  [unwired: 4 in, 7 out]
  "Stage Control Serial Error" <- w4
  n61 = node-c288() -> (w56:T35)  [unwired: 4 in]
  n62 = timed-loop "Run Scripts, including: stage motion" {
    tunnel: w4 -> [w218]
    tunnel: w1 -> [w219]
    tunnel: [w219] -> w58
    tunnel: [w218] -> w57
    timing: w56 -> [_]
    timing-out: [_] -> w55
    tunnel: w47 -> [w217]
    tunnel: w48 -> [w216]
    tunnel: w43 -> [w213]
    tunnel: w42 -> [w212]
    tunnel: w41 -> [w214]
    tunnel: w40 -> [w215]
    tunnel: w32 -> [w211]
    tunnel: w25 -> [w210]
    tunnel: w13 -> [w209]
    tunnel: w12 -> [w208]
    stop <- w220 stop-if-true
    n63 = node-c288() -> ()  [unwired: 1 in, 1 out]
    n64 = event shown="[13] \"Cal/Data Acq. Spot\": Value Change" {
      selector: _ -> [_ _ _ _ _ _ _ _ _ _ _ _ _ _ _ _ _ _ _ _ _ _ _ _ _ _ _]
      dyn-events: _ -> [_ _ _ _ _ _ _ _ _ _ _ _ _ _ _ _ _ _ _ _ _ _ _ _ _ _ _]
      timeout: _ -> [_ _ _ _ _ _ _ _ _ _ _ _ _ _ _ _ _ _ _ _ _ _ _ _ _ _ _]
      tunnel: ["Set Position" _ "Move to Position" _ _ _ _ _ _ "Read Harvard" _ _ _ _ _ _ _ _ "Force FB Data\nScript" _ _ "Take Stepping Data" _ "Take Detection Laser\nImage" _ _ _] -> _
      tunnel: [_ _ _ _ _ _ _ _ _ _ _ _ _ _ _ _ _ _ _ _ _ _ _ _ _ w1155 _] -> w220
      tunnel: w218 -> [w239 w247 w258 w271 w301 _ _ _ _ _ w438 w472 w498 w531 w633 w662 w794 w822 w853 _ _ _ _ _ _ _ _]
      tunnel: w219 -> [w240 w248 w259 w272 w302 _ _ _ _ _ w439 w473 w499 w532 w634 w663 w795 w823 w854 _ _ _ _ _ _ _ _]
      tunnel: w217 -> [_ _ _ _ _ _ _ _ _ w423 _ _ _ _ _ _ _ _ _ _ _ _ _ _ _ _ _]
      tunnel: w216 -> [_ _ _ _ _ _ _ _ _ w422 _ _ _ _ _ _ _ _ _ _ _ _ _ _ _ _ _]
      tunnel: w215 -> [_ _ _ _ _ _ _ _ _ _ _ _ _ _ _ _ _ _ _ _ _ _ _ _ _ _ _]
      tunnel: w214 -> [_ _ _ _ _ _ _ _ _ _ _ _ _ _ _ _ _ _ _ _ _ _ _ _ _ _ _]
      tunnel: w213 -> [_ _ _ _ _ _ _ _ _ _ _ _ _ _ _ _ _ _ _ _ _ _ _ _ _ _ _]
      tunnel: w212 -> [_ _ _ _ _ _ _ _ _ _ _ _ _ _ _ _ _ _ _ _ _ _ _ _ _ _ _]
      tunnel: w211 -> [_ _ _ _ _ w329 w336 w364 w383 _ _ _ _ _ _ _ _ _ _ _ _ _ _ _ _ w1154 _]
      tunnel: w210 -> [_ _ _ _ _ _ _ _ _ _ _ _ _ w524 _ _ _ _ _ _ _ _ _ _ w1021 _ _]
      tunnel: w209 -> [_ _ _ _ _ _ _ _ _ _ _ _ _ _ _ _ _ _ _ _ _ _ _ _ _ _ w1165]
      tunnel: w208 -> [_ _ _ _ _ _ _ _ _ _ _ _ _ _ _ _ _ _ _ _ _ _ _ _ _ _ w1160]
      event "Set Position", "Set Position 2", "Set Position 3", "Set Position 4", "Set Position 5", "Set Position 1", "Set Position 6": Value Change {